vi "UHR-Fleezers Control (host) - 12.2.vi"() -> ()   [LabVIEW 2014] (continued)
      }
    }
    n3142 = Unbundle By Name(w3932) -> ("Y"=w3935:dbl[])
    n3143 = Unbundle By Name(w3929) -> ("Y"=w3938:dbl[])
    n3144 = Subtract(x=w3935, y=w3933) -> (x-y=w3936:dbl[])
    n3145 = Subtract(x=w3938, y=w3931) -> (x-y=w3937:dbl[])
    n3146 = Multiply(x=w3937, y="T2 a_x (nm/V)") -> (x*y=w3739:dbl[])
    n3147 = Multiply(x="T1 a_x (nm/V)", y=w3936) -> (x*y=w3740:dbl[])
    n3148 = Not(x="Trap Trig. Fl.") -> (.not. x?=w3776:bool)
    n3149 = Multiply(x=w3959, y=-1.0) -> (x*y=w3940:waveform(dbl))
    n3150 = Subtract(x=w3740, y=w3739) -> (x-y=w3928:dbl[])
    n3151 = Unbundle By Name(w3959) -> ("Y"=w3902:dbl[])
    n3152 = Unbundle By Name(w3960) -> ("Y"=w3741:dbl[])
    n3153 = Negate(x=w3928) -> (-x=w3737:dbl[])
    n3154 = Build Array(w3960, w3940) -> (→"Force":waveform(dbl)[])
    n3155 = Subtract(x=w3737, y="Offset (nm)") -> (x-y=w3900:dbl[])
    n3156 = case shown="True" "Read Lateness and Rel Phase" {
      tunnel: w3757 -> [w4306 w4330]
      tunnel: w3756 -> [w4307 w4329]
      tunnel: [w4306 w4328] -> w3926
      tunnel: [w4307 w4327] -> w3925
      frame False {
      }
      frame True {
        n3157 = xnode "Read/Write Control"("FPGA VI Reference In"=w4330, "error in"=w4329) -> ("FPGA VI Reference Out"=w4328:T22, "error out"=w4327:errorcluster, "GI Relative phase"=→"GI relative phase":i16, "Relative phase"=→"Relative phase (AI1)":i16, "AI Late Counter"=→"Late Counter (AI1)":u8, "GI Late Counter"=→"GI Late Counter":u8, "MCL Late Counter"=→"MCL Late Counter":u8, "MCL Relative Phase"=→"Relative Phase (MCL)":i16, "APD Acq Relative Phase"=→"APD Acq Relative Phase":i16, "APD 1 Gate Relative Phase"=→"APD 1 Gate Relative Phase":i16, "APD 2 Gate Relative Phase"=→"APD 2 Gate Relative Phase":i16, "APD Acq Late Counter"=→"APD Acq Late Counter":u8, "APD 1 Gate Late Counter"=→"APD 1 Gate Late Counter":u8, "APD 2 Gate Late Counter"=→"APD 2 Gate Late Counter":u8, "Green FB Relative Phase"=→"Relative phase (Green FB)":i16, "GI Relative phase 2"=→"GI relative phase 2":i16, "GI Late Counter 2"=→"GI Late Counter 2":u8, "Trap Pos FIFO Timeout"=→"Trap Pos FIFO Timeout":u16, "Trap AI FIFO Timeout"=→"Trap AI FIFO Timeout":u16, "RI relative phase"=→"RI relative phase":i16, "RI late counter"=→"RI late counter":u8)
      }
    }
    n3158 = call-poly <vilib>:"Mean.vi"("X"=w3902) -> ("mean"=w3743:dbl)  [unwired: 1 out]
    "T2 X" <- w3743
    n3159 = Negate(x=w3902) -> (-x=w3903:dbl[])
    n3160 = call-poly <vilib>:"Mean.vi"("X"=w3741) -> ("mean"=w3744:dbl)  [unwired: 1 out]
    "T1 X" <- w3744
    n3161 = Negate(x=w3743) -> (-x=w3742:dbl)
    n3162 = Bundle By Name(cluster=w3932, "Y"=w3900) -> (w3877:waveform(dbl))
    "Bead Separation" <- w3877
    n3163 = Add(x=w3741, y=w3903) -> (x+y=w3904:dbl[])
    n3164 = Add(x=w3744, y=w3742) -> (x+y=w3946:dbl)
    n3165 = Subtract(x=w3744, y=w3742) -> (x-y=→"Difference":dbl)
    n3166 = Divide(x=w3904, y=2.0) -> (x/y=→"Vec Mean of T1 T2":dbl[])
    n3167 = Divide(x=w3946, y=2.0) -> (x/y=w3906:dbl)
    "Mean" <- w3906
    n3168 = feedback-in #27("Trap Trig. Fl.") -> ()
    n3169 = feedback #27("Trap Trig. Fl.") -> (w3774:bool)
    n3170 = And(x=w3776, y=w3774) -> (x .and. y?=w3775:bool)
    n3171 = case "If have just turned off triggering" shown="True" w3775 {
      tunnel: w3757 -> [_ w4136]
      tunnel: w3756 -> [_ w4135]
      frame False {
      }
      frame True {
        w4134 = FALSE ("FPGA Trap Trig")
        n3172 = xnode "Read/Write Control"("FPGA VI Reference In"=w4136, "error in"=w4135, "FPGA Trap Trig"=w4134) -> ("FPGA VI Reference Out"=w4133:T22, "error out"=w4132:errorcluster)
        n3173 = xnode "Read/Write Control"("FPGA VI Reference In"=w4133, "error in"=w4132, "TTrig?"=w4134) -> ()  [unwired: 2 out]
        n3174 = local write "Initializing"(FALSE ("Initializing")) -> ()
        n3175 = local write "Triggered"(FALSE ("Triggered")) -> ()
        n3176 = local write "Waiting"(FALSE ("Waiting")) -> ()
      }
    }
    n3177 = Not(x=w3774) -> (.not. x?=w3787:bool)
    n3178 = And(x="Trap Trig. Fl.", y=w3787) -> (x .and. y?=w3784:bool)
    n3179 = local read "Tether"() -> (w3907:bool)
    n3180 = Or(x=w3784, y="Reinitialize") -> (x .or. y?=w3770:bool)
    n3181 = feedback #28(w3780) -> (w3785:string)
    n3182 = Select(t=w3780, s=w3784, f=w3785) -> (s? t:f=w3779:string)
    n3183 = Select(t=w3780, s="Reinitialize", f=w3779) -> (s? t:f=w3778:string)
    n3184 = feedback #29(0) -> (w3782:i32)
    n3185 = feedback #30(w3900) -> (w3899:dbl[])
    n3186 = Build Array (concatenate)(w3900, w3899) -> (w3738:dbl[])
    n3187 = case "For determining if there is a tether still" shown="True" w3907 {
      tunnel: w3906 -> [_ w4260]
      frame False {
      }
      frame True {
        n3188 = Greater?(x="Lost Tether Alarm Threshold (pN)", y=w4260) -> (0:w4258:bool)
        n3189 = case shown="True" w4258 {
          frame False {
          }
          frame True {
            w4261 = TRUE
            w4265 = FALSE ("Multiple tether")
            w4266 = FALSE ("Value (Signaling)")
            n3190 = flat-sequence {
              frame #0 {
                # "stop only if saving"
                n3191 = local read "Saving..."() -> (w4278:bool)
                n3192 = And(x=w4278, y="TA Cancel Save?") -> (x .and. y?=w4277:bool)
                n3193 = local write "Stop Saving"(w4277) -> ()
              }
              frame #1 {
                n3194 = case shown="True" "TA Green Off?" {
                  frame False {
                  }
                  frame True {
                    w4281 = FALSE ("Fl. Triggered...")
                    n3195 = local write "Fl. Triggered..."(w4281) -> ()
                    n3196 = property on="Green ON/Interlacing" class="Bool (strict)"("Val(Sgnl)"=w4281) -> ()  [unwired: 2 in, 2 out]
                  }
                }
              }
            }
            n3197 = local read "Time tether formed"() -> (w4272:timestamp)
            n3198 = Get Date/Time In Seconds() -> (seconds since 1Jan1904=w4273:timestamp)
            n3199 = Subtract(x=w4273, y=w4272) -> (x-y=w4271:dbl)
            n3200 = Number To Decimal String(number=w4271) -> (decimal integer string=w4268:string)  [unwired: 1 out]
            n3201 = local read "Messages"() -> (w4275:string)
            n3202 = call <vilib>:"Beep.vi"("use system alert? (T)"=FALSE, "duration (msec)"=u32 200, "frequency (Hz)"=u32 200) -> ()  [unwired: 9 out]
            n3203 = Concatenate Strings("Lost tether (" ("Message to add"), w4268, " s)." ("string")) -> (w4270:string)
            n3204 = local write "Tether"(FALSE ("Tether")) -> ()
            n3205 = call "Update messages.vi"("Message to add"=w4270, "Old message string"=w4275) -> ("New message string"=w4274:string)
            n3206 = local write "Messages"(w4274) -> ()
            n3207 = local write "Pause dwell"(w4266) -> ()
            n3208 = property on="Fl. Triggered..." class="Bool (strict)"("Val(Sgnl)"=w4266) -> ()  [unwired: 2 in, 2 out]
            n3209 = local write "Dip for Protein"(w4266) -> ()
            n3210 = property on="Trap Pos. FB ON" class="Bool (strict)"("Val(Sgnl)"=w4266) -> ()  [unwired: 2 in, 2 out]
            n3211 = property on="Trap Trig. Fl." class="Bool (strict)"("Val(Sgnl)"=w4266) -> ()  [unwired: 2 in, 2 out]
            n3212 = local write "Multiple tether"(w4265) -> ()
            n3213 = local write "Bad fit"(w4265) -> ()
            n3214 = local write "Hysteresis"(w4265) -> ()
            n3215 = local write "Good tether"(w4265) -> ()
            n3216 = local write "Save scans"(w4261) -> ()
            n3217 = local write "Restart DMA? (AOD)"(w4261) -> ()
          }
        }
      }
    }
    n3218 = case "For triggering actions based on the trap position (e.g., turning the excitation laser on if trap under feedback moves so far)" shown="True" "Trap Trig. Fl." {
      tunnel: w3765 -> [_ w4149]
      tunnel: w3778 -> [_ w4148]
      tunnel: ["" ("t") w4147] -> w3786
      tunnel: w3770 -> [_ w4146]
      tunnel: [0 ("t") w4145] -> w3783
      tunnel: w3782 -> [_ w4144]
      tunnel: w3757 -> [_ w4143]
      tunnel: w3756 -> [_ w4142]
      frame False {
      }
      frame True {
        n3219 = case shown="\"Wait for trigger\"" w4148 {
          tunnel: w4149 -> [w4166 _ _ w4214]
          tunnel: [w4163 w4195 "" ("t") w4217] -> w4147
          tunnel: w4146 -> [_ _ _ w4205]
          tunnel: [w4162 w4192 0 ("t") w4206] -> w4145
          tunnel: w4144 -> [_ w4194 _ w4212]
          tunnel: w4143 -> [w4151 w4189 _ w4208]
          tunnel: w4142 -> [w4150 w4188 _ w4207]
          frame "Wait for trigger" {
            n3220 = local read "Trap Trig. (FPGA)"() -> (w4154:bool)
            n3221 = Subtract(x=w4166, y="Mean T1 Position\nto compare (nm)") -> (x-y=w4159:dbl[])
            n3222 = call <vilib>:"Std Deviation and Variance.vi"("X"=w4159) -> ("mean"=→"mean":dbl, "standard deviation"=→"standard\ndeviation":dbl)  [unwired: 1 in, 1 out]
            n3223 = Array Max & Min(array=w4159) -> (max value=→"max value":dbl, min value=→"min value":dbl)  [unwired: 2 out]
            n3224 = Greater?(x=w4159, y="Threshold (nm)") -> (0:w4169:bool[])
            n3225 = case shown="True" w4154 {
              tunnel: w4151 -> [_ w4175]
              tunnel: w4150 -> [_ w4174]
              tunnel: [FALSE ("TTrig?") w4173] -> w4157
              frame False {
              }
              frame True {
                n3226 = xnode "Read/Write Control"("FPGA VI Reference In"=w4175, "error in"=w4174) -> ("TTrig?"=w4173:bool)  [unwired: 2 out]
              }
            }
            n3227 = Or Array Elements(Boolean array=w4169) -> (logical OR=w4156:bool)
            n3228 = Select(t=w4157, s=w4154, f=w4156) -> (s? t:f=w4155:bool)
            n3229 = Not(x=w4154) -> (.not. x?=w4153:bool)
            n3230 = And(x=w4155, y=w4153) -> (x .and. y?=w4152:bool)
            n3231 = Select(t="Triggered", s=w4155, f="Wait for trigger") -> (s? t:f=w4163:string)
            n3232 = case shown="True" w4155 {
              tunnel: [0 0] -> w4162
              tunnel: w4151 -> [_ w4180]
              tunnel: w4150 -> [_ w4179]
              frame False {
                "Waiting" <- TRUE ("Waiting")
              }
              frame True {
                n3233 = xnode "Read/Write Control"("FPGA VI Reference In"=w4180, "error in"=w4179, "TTrig?"=FALSE) -> ()  [unwired: 2 out]
                n3234 = local read "Messages"() -> (w4183:string)
                n3235 = call <vilib>:"Beep.vi"() -> ()  [unwired: 12 in]
                n3236 = call "Update messages.vi"("Message to add"="Unwinding trigger.", "Old message string"=w4183) -> ("New message string"=w4184:string)
                n3237 = local write "Messages"(w4184) -> ()
                n3238 = local write "Waiting"(FALSE ("Waiting")) -> ()
                "Triggered" <- TRUE ("Triggered")
              }
            }
            n3239 = case "Only need to turn on laser if host triggered" shown="True" w4152 {
              frame False {
              }
              frame True {
                n3240 = property on="Green ON/Interlacing" class="Bool (strict)"("Val(Sgnl)"=TRUE ("Value (Signaling)")) -> ()  [unwired: 2 in, 2 out]
              }
            }
          }
          frame "Triggered" {
            n3241 = local read "Trap Trig. (FPGA)"() -> (w4191:bool)
            n3242 = Increment(x=w4194) -> (x+1=w4192:i32)
            n3243 = Greater Or Equal?(x=w4192, y="Fl. ON time (n)") -> (x >= y?=w4190:bool)
            n3244 = Select(t="Wait for trigger", s=w4190, f="Triggered" ("t")) -> (s? t:f=w4195:string)
            n3245 = And(x=w4190, y=w4191) -> (x .and. y?=w4187:bool)
            n3246 = case shown="True" w4187 {
              tunnel: w4189 -> [_ w4199]
              tunnel: w4188 -> [_ w4198]
              frame False {
              }
              frame True {
                n3247 = xnode "Read/Write Control"("FPGA VI Reference In"=w4199, "error in"=w4198, "FPGA Trap Trig"=TRUE) -> ()  [unwired: 2 out]
              }
            }
            n3248 = case shown="True" w4190 {
              frame False {
              }
              frame True {
                w4201 = FALSE ("Value (Signaling)")
                n3249 = local write "Triggered"(w4201) -> ()
                n3250 = local write "Waiting"(TRUE ("Waiting")) -> ()
                n3251 = property on="Green ON/Interlacing" class="Bool (strict)"("Val(Sgnl)"=w4201) -> ()  [unwired: 2 in, 2 out]
              }
            }
          }
          frame "Do nothing" {
          }
          frame "Initialize", Default {
            n3252 = Increment(x=w4212) -> (x+1=w4216:i32)
            n3253 = Select(t=1, s=w4205, f=w4216) -> (s? t:f=w4206:i32)
            n3254 = feedback #31(w4214) -> (w4220:dbl[])
            n3255 = Build Array (concatenate)(w4214, w4220) -> (w4213:dbl[])
            n3256 = Greater Or Equal?(x=w4206, y="Wait to get offset (n)") -> (x >= y?=w4209:bool)
            n3257 = Select(t=w4214, s=w4205, f=w4213) -> (s? t:f=w4215:dbl[])
            n3258 = feedback-in #31(w4215) -> ()
            n3259 = call-poly <vilib>:"Mean.vi"("X"=w4215) -> ("mean"=w4210:dbl)  [unwired: 1 out]
            n3260 = local write "Mean T1 Position\nto compare (nm)"(w4210) -> ()
            n3261 = case shown="True" w4205 {
              tunnel: w4208 -> [_ w4226]
              tunnel: w4207 -> [_ w4225]
              frame False {
              }
              frame True {
                w4222 = FALSE ("FPGA Trap Trig")
                n3262 = xnode "Read/Write Control"("FPGA VI Reference In"=w4226, "error in"=w4225, "FPGA Trap Trig"=w4222) -> ("FPGA VI Reference Out"=w4224:T22, "error out"=w4223:errorcluster)
                n3263 = xnode "Read/Write Control"("FPGA VI Reference In"=w4224, "error in"=w4223, "TTrig?"=w4222) -> ()  [unwired: 2 out]
              }
            }
            n3264 = Select(t="Wait for trigger", s=w4209, f="Initialize") -> (s? t:f=w4217:string)
            n3265 = case shown="True" w4209 {
              tunnel: w4210 -> [_ w4229]
              tunnel: w4208 -> [_ w4238]
              tunnel: w4207 -> [_ w4237]
              frame False {
                n3266 = local write "Waiting"(FALSE ("Waiting")) -> ()
                "Initializing" <- TRUE ("Initializing")
              }
              frame True {
                n3267 = local read "Threshold (nm)"() -> (w4241:dbl)
                n3268 = local read "AOM X Cal (nm/MHz)"() -> (w4240:dbl)
                n3269 = Add(x=w4229, y=w4241) -> (x+y=w4242:dbl)
                n3270 = Divide(x=w4242, y=w4240) -> (x/y=w4239:dbl)
                n3271 = call "IR AOM freq to word.vi"("Frequency In (MHz)"=w4239) -> ("Frequency Word Out (double)"=w4236:dbl)
                n3272 = local write "Initializing"(FALSE ("Initializing")) -> ()
                n3273 = local write "Waiting"(TRUE ("Waiting")) -> ()
                n3274 = To Quad Integer(1:w4236) -> (0:w4235:i64)
                n3275 = xnode "Read/Write Control"("FPGA VI Reference In"=w4238, "error in"=w4237, "FPGA TTrig Thresh"=w4235) -> ("FPGA VI Reference Out"=w4232:T22, "error out"=w4231:errorcluster)
                n3276 = xnode "Read/Write Control"("FPGA VI Reference In"=w4232, "error in"=w4231, "FPGA Trap Trig"=TRUE) -> ()  [unwired: 2 out]
              }
            }
          }
        }
      }
    }
    n3277 = feedback-in #28(w3786) -> ()
    n3278 = feedback-in #29(w3783) -> ()
    n3279 = Split 1D Array(array=w3738, index=w3800) -> (first subarray=w3896:dbl[])  [unwired: 1 out]
    n3280 = feedback-in #30(w3896) -> ()
    n3281 = call-poly <vilib>:"Mean.vi"("X"=w3896) -> ("mean"=w3895:dbl)  [unwired: 1 out]
    "Bead Mean (nm)" <- w3895
    n3282 = Subtract(x=w3896, y=w3895) -> (x-y=w3894:dbl[])
    n3283 = Square(x=w3894) -> (x^2=w3893:dbl[])
    n3284 = call-poly <vilib>:"Mean.vi"("X"=w3893) -> ("mean"=w3892:dbl)  [unwired: 1 out]
    n3285 = Square Root(x=w3892) -> (sqrt(x)=w3891:dbl)
    n3286 = Multiply(x=10.0, y=w3891) -> (x*y=→"RMS (Å)":dbl)
    n3287 = xnode ("Read/Write Control")("FPGA VI Reference In"=w3926, "error in"=w3925) -> ("FPGA VI Reference Out"=w3768:T22, "error out"=w3767:errorcluster, "AI2 Y Sum Set 1"=w4021:i16, "AI2 Y Sum Set 2"=w4020:i16, "AI1 X Set 1"=w3828:fxp<+/-,16,1>, "AI1 X Set 2"=w3827:fxp<+/-,16,1>, "Trap Pos FB Int Signal"=→"Trap Pos FB Int Signal":fxp<+/-,24,9>, "Trap Pos FB Int-Norm Signal"=→"Trap Pos FB Int-Norm Signal":fxp<+/-,16,1>, "Trap Pos FB Action"=w3821:i64, "Scanning"=→"AOD Scanning":bool, "Scan I"=→"AOD Scan I":u64, "Scanning MCL"=w4023:bool, "Scan I (MCL)"=→"MCL Scan I":u64, "Green FB Sum"=w3963:i16, "Trap Pos FB Action"=w3755:i64, "Wiggling 1"=→"Wiggling T1":bool, "TTrig Fin Thresh"=w3751:i64, "Wiggling 2"=→"Wiggling T2":bool, "Red FB Sum"=w3718:i16)  [unwired: 2 out]
    "MCL Scanning" <- w4023
    "Trap Pos FB Action" <- w3821
    n3288 = local read "FB Trig Integrate"() -> (w3749:u32)
    n3289 = Divide(x=w3963, y=3276.7) -> (x/y=w3717:dbl)
    "Green laser intensity (V)" <- w3717
    n3290 = Divide(x=w3718, y=3276.7) -> (x/y=w3716:dbl)
    "Red laser intensity (V)" <- w3716
    n3291 = Divide(x=w3755, y=w3749) -> (x/y=w3748:dbl)
    "TTrig Sig (Int)" <- w3748
    n3292 = Divide(x=w3751, y=w3749) -> (x/y=w3746:dbl)
    "TTrig Fin Thresh (Int)" <- w3746
    n3293 = local read "AOM X Cal (nm/MHz)"() -> (w3754:dbl)
    n3294 = local read "AI2 (V)"() -> (w4022:cluster{"Set 1":dbl, "Set 2":dbl})
    n3295 = Bundle By Name(cluster=w4022, "Set 1"=w4021, "Set 2"=w4020) -> (w4018:cluster{"Set 1":dbl, "Set 2":dbl})
    n3296 = Divide(x=w3821, y=327.67) -> (x/y=w3733:dbl)
    n3297 = local read "Trap X (AI1)"() -> (w3841:T10)
    n3298 = Bundle(w3717, w3716) -> (→"Excitation laser intensities plot":cluster{dbl, dbl})  [unwired: 1 in]
    n3299 = call "IR AOM word double to freq.vi"("Frequency Word In (double)"=w3746) -> ("Frequency Out (MHz)"=w3745:dbl)
    n3300 = call "IR AOM word double to freq.vi"("Frequency Word In (double)"=w3748) -> ("Frequency Out (MHz)"=w3747:dbl)
    n3301 = Divide(x=w4018, y=3276.7) -> (x/y=w4017:cluster{"Set 1":dbl, "Set 2":dbl})
    n3302 = Multiply(x=w3747, y=w3754) -> (x*y=w3753:dbl)
    "TTrig Sig (nm)" <- w3753
    n3303 = Multiply(x=w3745, y=w3754) -> (x*y=w3752:dbl)
    "TTrig Fin Thresh (nm)" <- w3752
    n3304 = local write "AI2 (V)"(w4017) -> ()
    n3305 = local read "Trap Pos. FB Range"() -> (w3732:T12)
    n3306 = Bundle(cluster=w3841, "Trap 1"=w3828, "Trap 2"=w3827) -> (→"Trap X (AI1)":T10)
    n3307 = Bundle(w3753, w3752) -> (→"TTrig":cluster{dbl, dbl})  [unwired: 1 in]
    n3308 = Unbundle(w3732) -> ("output high"=w3731:fxp<+/-,64,32>)  [unwired: 1 out]
    n3309 = Divide(x=w3733, y=w3731) -> (x/y=→"Action (%)":dbl)
    n3310 = flat-sequence "To save data" {
      tunnel: [w5105] -> w4040
      tunnel: [w5106] -> w4039
      tunnel: w3993 -> [w5078]
      tunnel: w3773 -> [w5103]
      tunnel: ["Save Calibration"] -> w4014
      tunnel: w4011 -> [w5102]
      tunnel: [w5096] -> w4010
      tunnel: [w5093] -> w4009
      tunnel: [w5090] -> w4008
      tunnel: w3992 -> [w5092]
      tunnel: w3910 -> [w5086]
      tunnel: [w5086] -> w3909
      tunnel: ["Start Saving"] -> w3879
      tunnel: [w5080] -> w3813
      tunnel: [w5079] -> w3812
      tunnel: [w5075] -> w3697
      tunnel: w4040 -> [w5380]
      tunnel: w4039 -> [w5379]
      tunnel: w3814 -> [w5378]
      tunnel: w4014 -> [w5377]
      tunnel: w4010 -> [w5375]
      tunnel: w4009 -> [w5374]
      tunnel: w4008 -> [w5373]
      tunnel: w3888 -> [w5372]
      tunnel: w3919 -> [w5371]
      tunnel: w3909 -> [w5370]
      tunnel: w3879 -> [w5369]
      tunnel: w3877 -> [w5368]
      tunnel: w3855 -> [w5367]
      tunnel: w3813 -> [w5366]
      tunnel: w3812 -> [w5365]
      tunnel: w3811 -> [w5364]
      tunnel: w3734 -> [w5363]
      tunnel: w3697 -> [w5362]
      frame #0 {
        n3311 = Or(x="Save N Sets", y="Start Saving") -> (x .or. y?=w5087:bool)
        n3312 = To Double Precision Float(number=w5102) -> (double precision float=w5097:dbl)
        n3313 = Build Array(w5087, "Save Calibration", w5078, w5092) -> (w5101:bool[])
        n3314 = Compound Arithmetic op=OR("Save Calibration", w5078, w5087, w5092) -> (w5104:bool)
        n3315 = Boolean Array To Number(Boolean array=w5101) -> (number=w5099:u32)
        n3316 = feedback #32(FALSE ("Save APD Data\nwith Trap Data")) -> (w5081:bool)
        n3317 = feedback #33(refnum<k0> refnum) -> (w5076:refnum<file>)
        n3318 = feedback #34(refnum<k0> refnum) -> (w5107:refnum<file>)
        n3319 = feedback #35(refnum<k0> refnum) -> (w5083:refnum<file>)
        n3320 = feedback #36(FALSE ("Save APD Data\nwith Trap Data")) -> (w5091:bool)
        n3321 = feedback #37(refnum<k0> refnum) -> (w5094:refnum<file>)
        n3322 = feedback #38(0) -> (w5109:i32)
        n3323 = feedback #39() -> (w5098:u32)  [unwired: 1 out]
        n3324 = case shown="True" w5104 {
          tunnel: [w5117 1] -> w5105
          tunnel: w5109 -> [w5119 _]
          tunnel: [w5118 w5139] -> w5106
          tunnel: w5107 -> [w5118 _]
          tunnel: w5103 -> [_ w5159]
          tunnel: w5097 -> [_ w5157]
          tunnel: w5099 -> [_ w5160]
          tunnel: [w5116 w5138] -> w5096
          tunnel: w5098 -> [w5116 _]
          tunnel: [w5115 w5136] -> w5093
          tunnel: w5094 -> [w5115 _]
          tunnel: [w5114 w5135] -> w5090
          tunnel: w5091 -> [w5114 _]
          tunnel: "Start Saving" -> [_ w5133]
          tunnel: w5086 -> [_ w5132]
          tunnel: [w5113 w5124] -> w5079
          tunnel: w5083 -> [w5113 _]
          tunnel: [w5112 w5122] -> w5080
          tunnel: w5081 -> [w5112 _]
          tunnel: w5076 -> [w5111 _]
          tunnel: [w5111 w5121] -> w5075
          frame False {
            n3325 = Increment(x=w5119) -> (x+1=w5117:i32)
          }
          frame True {
            w5129 = FALSE ("Start Saving")
            w5134 = 9.0  # File Version
            w5142 = FALSE ("prepend array or string size? (T)")
            w5140 = T29."big-endian, network order" ("byte order (0:big-endian, network order)")
            n3326 = local read "BD 1 Frequency 1 (MHz)"() -> (w5156:dbl)
            n3327 = local read "BD 2 Frequency 1 (MHz)"() -> (w5155:dbl)
            n3328 = local read "BD 1 Frequency 2 (MHz)"() -> (w5154:dbl)
            n3329 = local read "BD 2 Frequency 2 (MHz)"() -> (w5153:dbl)
            n3330 = local read "BD 1 Frequency 3 (MHz)"() -> (w5152:dbl)
            n3331 = local read "BD 2 Frequency 3 (MHz)"() -> (w5151:dbl)
            n3332 = Array Size(array=w5132) -> (size(s)=w5131:i32)
            n3333 = To Double Precision Float(number=w5131) -> (double precision float=w5130:dbl)
            n3334 = Build Array("Save APD Data\nwith Trap Data", "Save Trap Pos. Data") -> (w5126:bool[])
            n3335 = Boolean Array To Number(Boolean array=w5126) -> (number=w5125:u32)
            n3336 = Build Array(w5156, w5155, w5154, w5153, w5152, w5151) -> (w5150:dbl[])
            n3337 = case shown="4" w5160 {
              tunnel: w5159 -> [w5261 w5284 w5301 w5340]
              tunnel: w5130 -> [w5266 w5291 w5321 w5359]
              tunnel: w5157 -> [w5265 w5290 w5320 w5358]
              tunnel: [w5262 w5286 w5312 w5350] -> w5148
              tunnel: [w5254 "Cal sets to save" w5302 w5341] -> w5138
              tunnel: w5150 -> [w5263 w5287 w5314 w5352]
              tunnel: "Save APD Data\nwith Trap Data" -> [w5260 _ w5298 w5338]
              tunnel: [w5260 FALSE ("Save APD Data\nwith Trap Data") w5298 w5338] -> w5135
              tunnel: w5134 -> [w5257 w5281 w5296 w5336]
              tunnel: w5133 -> [w5256 _ _ _]
              tunnel: [w5243 "Active cal?" w5295 w5326] -> w5122
              tunnel: "Save Trap Pos. Data" -> [w5243 _ w5295 w5326]
              tunnel: w5125 -> [w5248 _ w5294 w5325]
              tunnel: [w5243 w5275 w5293 w5324] -> w5120
              frame 1, Default {
                # "timeseries"
                n3338 = case shown="True" "Profile" {
                  tunnel: [w5269 w5273] -> w5252
                  tunnel: [w5269 w5272] -> w5251
                  tunnel: [w5269 w5271] -> w5250
                  tunnel: [w5269 w5270] -> w5249
                  frame False {
                    w5269 = 0.0 ("f")
                  }
                  frame True {
                    n3339 = local read "Current Position"() -> (w5274:cluster{dbl, dbl, dbl})
                    n3340 = local read "Y change (mm)"() -> (w5270:dbl)
                    n3341 = Unbundle(w5274) -> (w5273:dbl, w5272:dbl, w5271:dbl)
                  }
                }
                n3342 = local read "Save ave N"() -> (w5268:dbl)
                n3343 = Multiply(x=w5268, y=w5261) -> (x*y=w5267:dbl)
                n3344 = To Double Precision Float(number=w5248) -> (double precision float=w5259:dbl)
                n3345 = Select(t=4.0, s="Profile", f=0.0) -> (s? t:f=w5244:dbl)
                n3346 = Build Array(w5257, w5261, w5267, w5266, w5265, w5244) -> (w5264:dbl[])
                n3347 = Build Array(w5259, w5252, w5251, w5250, w5249) -> (w5258:dbl[])
                n3348 = Select(t=u32 4000000000, s=w5256, f="N sets to save") -> (s? t:f=w5254:u32)
                n3349 = Build Array (concatenate)(w5264, w5263, w5258) -> (w5262:dbl[])
              }
              frame 2 {
                w5275 = FALSE
                w5283 = 0.0 ("f")
                # "If doing active calibration,\nalso save trap position file"
                # "calibration"
                n3350 = property on="Wiggle" class="Bool (strict)"("Val(Sgnl)"="Active cal?") -> ()  [unwired: 2 in, 2 out]
                n3351 = Select(t=2.0, s="Active cal?", f=0.0) -> (s? t:f=w5277:dbl)
                n3352 = Build Array(w5277, w5283, w5283, w5283, w5283) -> (w5282:dbl[])
                n3353 = Build Array(w5281, w5284, w5284, w5291, w5290, 1.0 ("t")) -> (w5288:dbl[])
                n3354 = local write "Saving Move"(w5275) -> ()
                n3355 = Build Array (concatenate)(w5288, w5287, w5282) -> (w5286:dbl[])
                "Calibrating..." <- TRUE ("Calibrating...")
              }
              frame 4 {
                w5293 = FALSE
                w5299 = 0.0 ("f")
                # "scan dir (x/y = 0/1)"
                # "cycles/step"
                # "n scans (f/b)"
                # "steps"
                # "freq. range"
                # "AOD raster scan"
                n3356 = local read "Number of F/B Scans (AOD)"() -> (w5306:u16)
                n3357 = local read "Cycles/step (AOD)"() -> (w5308:u64)
                n3358 = local read "Scan Range (MHz)"() -> (w5311:dbl)
                n3359 = local read "Scan steps (AOD)"() -> (w5310:u64)
                n3360 = local read "Scan BD"() -> (w5318:bool)
                n3361 = local read "Save ave N"() -> (w5323:dbl)
                n3362 = Boolean To (0,1)(Boolean=w5318) -> (0, 1=w5317:i16)
                n3363 = To Double Precision Float(number=w5306) -> (double precision float=w5305:dbl)
                n3364 = To Double Precision Float(number=w5310) -> (double precision float=w5309:dbl)
                n3365 = To Double Precision Float(number=w5308) -> (double precision float=w5307:dbl)
                n3366 = To Double Precision Float(number=w5317) -> (double precision float=w5316:dbl)
                n3367 = Multiply(x=w5323, y=w5301) -> (x*y=w5322:dbl)
                n3368 = To Double Precision Float(number=w5294) -> (double precision float=w5300:dbl)
                n3369 = Build Array(w5300, w5299, w5299, w5299, w5299) -> (w5297:dbl[])
                n3370 = local read "N sets should be saved"() -> (w5303:dbl)
                n3371 = local write "Raster Scanning..."(w5293) -> ()
                n3372 = Build Array(w5316, w5311, w5309, w5307, w5305) -> (w5313:dbl[])
                n3373 = Build Array(w5296, w5301, w5322, w5321, w5320, 2.0 ("t")) -> (w5315:dbl[])
                n3374 = local write "Saving Move"(w5293) -> ()
                n3375 = Round Toward +Infinity(x=w5303) -> (ceil(x): smallest int >= x=w5304:dbl)
                n3376 = Build Array (concatenate)(w5315, w5314, w5297, w5313) -> (w5312:dbl[])
                n3377 = To Unsigned Long Integer(number=w5304) -> (unsigned 32bit integer=w5302:u32)
              }
              frame 8 {
                w5324 = FALSE
                w5333 = 0.0 ("f")
                # "MCL raster scan"
                n3378 = local read "Number of scans (MCL)"() -> (w5328:u64)
                n3379 = local write "Saving Move"(w5324) -> ()
                n3380 = local read "Scan lines (y)"() -> (w5327:u64)
                n3381 = local read "2D or 1D Scan"() -> (w5330:bool)
                n3382 = local read "Scan Range (V)\n(of steps)"() -> (w5349:dbl)
                n3383 = local read "Fast Scan Dir"() -> (w5356:bool)
                n3384 = local read "Cycles/step (MCL)"() -> (w5346:u64)
                n3385 = local read "Scan steps (MCL)"() -> (w5348:u64)
                n3386 = Select(t=w5327, s=w5330, f=w5328) -> (s? t:f=w5329:u64)
                n3387 = Boolean To (0,1)(Boolean=w5330) -> (0, 1=w5332:i16)
                n3388 = local read "Save ave N"() -> (w5361:dbl)
                n3389 = local read "Initial X"() -> (w5335:dbl)
                n3390 = local read "Initial Y"() -> (w5334:dbl)
                n3391 = To Double Precision Float(number=w5332) -> (double precision float=w5331:dbl)
                n3392 = Boolean To (0,1)(Boolean=w5356) -> (0, 1=w5355:i16)
                n3393 = To Double Precision Float(number=w5329) -> (double precision float=w5344:dbl)
                n3394 = To Double Precision Float(number=w5348) -> (double precision float=w5347:dbl)
                n3395 = To Double Precision Float(number=w5346) -> (double precision float=w5345:dbl)
                n3396 = To Double Precision Float(number=w5355) -> (double precision float=w5354:dbl)
                n3397 = Multiply(x=w5361, y=w5340) -> (x*y=w5360:dbl)
                n3398 = To Double Precision Float(number=w5325) -> (double precision float=w5339:dbl)
                n3399 = local read "N sets should be saved (MCL)"() -> (w5342:dbl)
                n3400 = Build Array(w5339, w5331, w5333, w5333, w5333) -> (w5337:dbl[])
                n3401 = Build Array(w5354, w5349, w5347, w5345, w5344, w5335, w5334) -> (w5351:dbl[])
                n3402 = Build Array(w5336, w5340, w5360, w5359, w5358, 3.0 ("t")) -> (w5353:dbl[])
                n3403 = Round Toward +Infinity(x=w5342) -> (ceil(x): smallest int >= x=w5343:dbl)
                n3404 = Build Array (concatenate)(w5353, w5352, w5337, w5351) -> (w5350:dbl[])
                n3405 = To Unsigned Long Integer(number=w5343) -> (unsigned 32bit integer=w5341:u32)
              }
            }
            n3406 = local read "Index"() -> (w5165:dbl)
            n3407 = call "Create new save file.vi"("Insert"="", "Ext"=".dat", "Index In"=w5165) -> ("Path Out"=w5123:path, "Index Out"=w5137:dbl)
            n3408 = case shown="True" w5120 {
              tunnel: w5123 -> [_ w5172]
              tunnel: [refnum<k0> refnum w5170] -> w5121
              frame False {
              }
              frame True {
                n3409 = Path To String(path=w5172) -> (string=w5181:string)
                n3410 = Get Date/Time In Seconds() -> (seconds since 1Jan1904=w5191:timestamp)
                n3411 = String Length(string=w5181) -> (length=w5186:i32)
                n3412 = Subtract(x=w5186, y=4) -> (x-y=w5185:i32)
                n3413 = String Subset(string=w5181, length (rest)=w5185) -> (substring=w5183:string)  [unwired: 1 in]
                n3414 = call <vilib>:"Space Constant.vi"() -> ("String"=w5187:string)
                n3415 = Format Date/Time String(time format string (%c)="%H:%M:%S%3u", seconds (now)=w5191, UTC format=TRUE) -> (date/time string=w5188:string)
                n3416 = Concatenate Strings(w5183, "_stagetime.txt") -> (w5182:string)
                n3417 = String To Path(string=w5182) -> (path=w5179:path)
                n3418 = Open/Create/Replace File(file path (use dialog)=w5179, operation (0:open)=T30."create", access (0:read/write)=enum16{"read/write", "read-only", "write-only"}."write-only") -> (refnum out=w5178:refnum<file>, error out=w5175:errorcluster)  [unwired: 3 in, 1 out]
                n3419 = Deny Access(4:w5175, 7:w5178) -> (3:w5177:refnum<file>)  [unwired: 1 in, 1 out]
                n3420 = local read "Raster Scanning..."() -> (w5194:bool)
                n3421 = Concatenate Strings(w5188, w5187, "start", "\r\n") -> (w5176:string)
                n3422 = local read "Calibrating..."() -> (w5193:bool)
                n3423 = local write "Move Time"(w5188) -> ()
                n3424 = Write to Text File(file (use dialog)=w5177, text=w5176) -> (refnum out=w5170:refnum<file>)  [unwired: 2 in, 2 out]
                n3425 = Or(x=w5194, y=w5193) -> (x .or. y?=w5196:bool)
                n3426 = Not(x=w5196) -> (.not. x?=w5195:bool)
                n3427 = local write "Saving Move"(w5195) -> ()
              }
            }
            n3428 = local write "Save Calibration"(w5129) -> ()
            n3429 = local write "Start Saving"(w5129) -> ()
            n3430 = local write "Save file name"(w5123) -> ()
            n3431 = local write "Index"(w5137) -> ()
            n3432 = local write "Save index"(w5137) -> ()
            n3433 = Array Size(array=w5148) -> (size(s)=w5149:i32)
            n3434 = Open/Create/Replace File(file path (use dialog)=w5123, operation (0:open)=T30."create", access (0:read/write)=enum16{"read/write", "read-only", "write-only"}."write-only") -> (refnum out=w5162:refnum<file>)  [unwired: 1 in, 4 out]
            n3435 = local write "Saving..."(TRUE ("Saving...")) -> ()
            n3436 = To Double Precision Float(number=w5149) -> (double precision float=w5147:dbl)
            n3437 = String Length(string="Comment (data description)") -> (length=w5145:i32)
            n3438 = To Double Precision Float(number=w5145) -> (double precision float=w5144:dbl)
            n3439 = Deny Access(7:w5162) -> (3:w5161:refnum<file>)  [unwired: 1 in, 2 out]
            n3440 = Build Array (concatenate)(w5147, w5148, w5144) -> (w5146:dbl[])
            n3441 = case "If fluorescence data to be saved" shown="True" w5135 {
              tunnel: w5123 -> [_ w5242]
              tunnel: [refnum<k0> refnum w5222] -> w5136
              frame False {
              }
              frame True {
                w5221 = 0.0
                n3442 = local read "APD Integration Time (s)"() -> (w5227:dbl)
                n3443 = local read "N APD Samp/step"() -> (w5220:dbl)
                n3444 = Path To String(path=w5242) -> (string=w5241:string)
                n3445 = String Length(string=w5241) -> (length=w5240:i32)
                n3446 = Subtract(x=w5240, y=4) -> (x-y=w5238:i32)
                n3447 = String Subset(string=w5241, length (rest)=w5238) -> (substring=w5237:string)  [unwired: 1 out]
                n3448 = Build Array(w5227, w5220, w5221, w5221, w5221, w5221, w5221, w5221) -> (w5224:dbl[])
                n3449 = Concatenate Strings(w5237, "_fl.dat" ("string")) -> (w5235:string)
                n3450 = Array Size(array=w5224) -> (size(s)=w5226:i32)
                n3451 = String To Path(string=w5235) -> (path=w5231:path)
                n3452 = Open/Create/Replace File(file path (use dialog)=w5231, operation (0:open)=T30."create", access (0:read/write)=enum16{"read/write", "read-only", "write-only"}."write-only") -> (refnum out=w5232:refnum<file>)  [unwired: 1 in, 4 out]
                n3453 = Deny Access(7:w5232) -> (3:w5228:refnum<file>)  [unwired: 1 in, 2 out]
                n3454 = To Double Precision Float(number=w5226) -> (double precision float=w5225:dbl)
                n3455 = Build Array (concatenate)(w5225, w5224) -> (w5223:dbl[])
                n3456 = Write to Binary File(file (use dialog)=w5228, data=w5223, 5:FALSE ("prepend array or string size? (T)"), 9:T29."big-endian, network order" ("byte order (0:big-endian, network order)")) -> (refnum out=w5222:refnum<file>)  [unwired: 1 in, 3 out]
              }
            }
            n3457 = case shown="True" w5122 {
              tunnel: w5123 -> [_ w5204]
              tunnel: [refnum<k0> refnum w5203] -> w5124
              frame False {
              }
              frame True {
                w5199 = 0.0 ("element")
                n3458 = Path To String(path=w5204) -> (string=w5218:string)
                n3459 = Build Array(w5199, w5199, w5199, w5199, w5199, w5199, w5199, w5199) -> (w5200:dbl[])
                n3460 = String Length(string=w5218) -> (length=w5217:i32)
                n3461 = Subtract(x=w5217, y=4) -> (x-y=w5215:i32)
                n3462 = Array Size(array=w5200) -> (size(s)=w5202:i32)
                n3463 = String Subset(string=w5218, length (rest)=w5215) -> (substring=w5214:string)  [unwired: 1 out]
                n3464 = To Double Precision Float(number=w5202) -> (double precision float=w5201:dbl)
                n3465 = Concatenate Strings(w5214, "_pos.dat" ("string")) -> (w5212:string)
                n3466 = Build Array (concatenate)(w5201, w5200) -> (w5198:dbl[])
                n3467 = String To Path(string=w5212) -> (path=w5208:path)
                n3468 = Open/Create/Replace File(file path (use dialog)=w5208, operation (0:open)=T30."create", access (0:read/write)=enum16{"read/write", "read-only", "write-only"}."write-only") -> (refnum out=w5209:refnum<file>)  [unwired: 1 in, 4 out]
                n3469 = Deny Access(7:w5209) -> (3:w5205:refnum<file>)  [unwired: 1 in, 2 out]
                n3470 = Write to Binary File(file (use dialog)=w5205, data=w5198, 5:FALSE ("prepend array or string size? (T)"), 9:T29."big-endian, network order" ("byte order (0:big-endian, network order)")) -> (refnum out=w5203:refnum<file>)  [unwired: 1 in, 3 out]
              }
            }
            n3471 = Write to Binary File(file (use dialog)=w5161, data=w5146, 5:w5142, 9:w5140) -> (refnum out=w5143:refnum<file>)  [unwired: 1 in, 3 out]
            n3472 = Write to Binary File(file (use dialog)=w5143, data="Comment (data description)", 5:w5142, 9:w5140) -> (refnum out=w5139:refnum<file>)  [unwired: 1 in, 3 out]
          }
        }
        n3473 = feedback-in #32(w5080) -> ()
        n3474 = feedback-in #33(w5075) -> ()
        n3475 = feedback-in #34(w5106) -> ()
        n3476 = feedback-in #35(w5079) -> ()
        n3477 = feedback-in #36(w5090) -> ()
        n3478 = feedback-in #37(w5093) -> ()
        n3479 = feedback-in #38(w5105) -> ()
        n3480 = feedback-in #39(w5096) -> ()
      }
      frame #1 {
        n3481 = local read "Saving..."() -> (w5376:bool)
        n3482 = case shown="True" w5376 {
          tunnel: w5380 -> [_ w5393]
          tunnel: w5379 -> [_ w5406]
          tunnel: w5378 -> [_ w5402]
          tunnel: w5377 -> [_ w5401]
          tunnel: w5375 -> [_ w5382]
          tunnel: w5374 -> [_ w5396]
          tunnel: w5373 -> [_ w5395]
          tunnel: w5372 -> [_ w5394]
          tunnel: w5371 -> [_ w5392]
          tunnel: w5370 -> [_ w5390]
          tunnel: w5369 -> [_ w5389]
          tunnel: w5368 -> [_ w5388]
          tunnel: w5367 -> [_ w5387]
          tunnel: w5366 -> [_ w5386]
          tunnel: w5365 -> [_ w5385]
          tunnel: w5364 -> [_ w5384]
          tunnel: w5363 -> [_ w5383]
          tunnel: w5362 -> [_ w5381]
          frame False {
          }
          frame True {
            n3483 = Multiply(x=w5393, y=w5392) -> (x*y=→"Time (s)":dbl)
            n3484 = Less Or Equal?(x=w5393, y=w5382) -> (x <= y?=w5404:bool)
            n3485 = Or(x="Stop Saving", y="Abort save 2") -> (x .or. y?=w5397:bool)
            n3486 = Not(x=w5397) -> (.not. x?=w5405:bool)
            n3487 = And(x=w5404, y=w5405) -> (x .and. y?=w5403:bool)
            n3488 = case shown="False" w5403 {
              tunnel: w5406 -> [w5416 w5503]
              tunnel: [0.0 w5506] -> w5400
              tunnel: w5393 -> [_ w5504]
              tunnel: w5382 -> [_ w5505]
              tunnel: w5402 -> [_ w5500]
              tunnel: w5401 -> [_ _]
              tunnel: w5396 -> [w5414 w5493]
              tunnel: w5395 -> [w5413 w5494]
              tunnel: w5394 -> [_ w5492]
              tunnel: w5390 -> [_ w5491]
              tunnel: w5389 -> [_ w5435]
              tunnel: w5388 -> [_ w5484]
              tunnel: w5387 -> [_ w5462]
              tunnel: w5386 -> [w5411 w5444]
              tunnel: w5385 -> [w5412 w5443]
              tunnel: w5384 -> [_ w5440]
              tunnel: w5383 -> [_ w5438]
              tunnel: w5381 -> [w5409 w5430]
              frame False {
                w5407 = FALSE
                n3489 = Close File(refnum=w5416) -> ()  [unwired: 1 in, 2 out]
                n3490 = case shown="True" w5413 {
                  tunnel: w5414 -> [_ w5428]
                  frame False {
                  }
                  frame True {
                    n3491 = Close File(refnum=w5428) -> ()  [unwired: 1 in, 2 out]
                  }
                }
                n3492 = case shown="True" w5411 {
                  tunnel: w5412 -> [_ w5427]
                  frame False {
                  }
                  frame True {
                    n3493 = Close File(refnum=w5427) -> ()  [unwired: 1 in, 2 out]
                  }
                }
                n3494 = local read "Saving Move"() -> (w5408:bool)
                n3495 = case shown="True" w5408 {
                  tunnel: w5409 -> [_ w5419]
                  frame False {
                  }
                  frame True {
                    n3496 = Get Date/Time In Seconds() -> (seconds since 1Jan1904=w5424:timestamp)
                    n3497 = call <vilib>:"Space Constant.vi"() -> ("String"=w5422:string)
                    n3498 = Format Date/Time String(time format string (%c)="%H:%M:%S%3u", seconds (now)=w5424, UTC format=TRUE) -> (date/time string=w5418:string)
                    n3499 = Concatenate Strings(w5418, w5422, "end") -> (w5420:string)
                    n3500 = Write to Text File(file (use dialog)=w5419, text=w5420) -> (refnum out=w5426:refnum<file>)  [unwired: 2 in, 2 out]
                    n3501 = Close File(refnum=w5426) -> ()  [unwired: 1 in, 2 out]
                    n3502 = property on="Move Time" class="Str"("Value"=w5418) -> ()  [unwired: 2 in, 2 out]
                    n3503 = local write "Saving Move"(FALSE) -> ()
                  }
                }
                n3504 = call <vilib>:"Beep.vi"() -> ()  [unwired: 3 in, 9 out]
                n3505 = local write "Raster Scanning..."(w5407) -> ()
                n3506 = local write "Calibrating..."(w5407) -> ()
                n3507 = property on="Abort wiggle" class="Bool (strict)"("Val(Sgnl)"=TRUE) -> ()  [unwired: 2 in, 2 out]
                n3508 = local write "Stop Saving"(w5407) -> ()
                "Saving..." <- w5407
              }
              frame True {
                n3509 = local read "Calibrating..."() -> (w5495:bool)
                n3510 = case "Write fl. data" shown="True" w5494 {
                  tunnel: w5493 -> [_ w5535]
                  tunnel: w5492 -> [_ w5534]
                  frame False {
                  }
                  frame True {
                    n3511 = Write to Binary File(file (use dialog)=w5535, data=w5534, 5:FALSE ("prepend array or string size? (T)"), 9:T29."big-endian, network order" ("byte order (0:big-endian, network order)")) -> ()  [unwired: 1 in, 4 out]
                  }
                }
                n3512 = Greater?(x="Save ave N", y=1.0) -> (0:w5498:bool)
                n3513 = Not(x=w5495) -> (.not. x?=w5497:bool)
                n3514 = local read "Saving Move"() -> (w5429:bool)
                n3515 = And(x=w5497, y=w5498) -> (x .and. y?=w5441:bool)
                n3516 = case shown="True" w5441 {
                  tunnel: w5440 -> [w5515 w5526]
                  tunnel: [w5515 w5518] -> w5439
                  tunnel: "Save ave N" -> [_ w5519]
                  frame False {
                  }
                  frame True {
                    w5516 = 2 ("dimension size")
                    n3517 = Array Size(array=w5526) -> (size(s)=w5520:i32)
                    n3518 = Divide(x=w5520, y=w5516) -> (x/y=w5524:dbl)
                    n3519 = Reshape Array(w5526, w5524, w5516) -> (w5525:u64[][])
                    n3520 = Transpose 2D Array(2D array=w5525) -> (transposed array=w5523:u64[][])
                    n3521 = for {
                      tunnel: w5523 -> [w5528] mode=indexing
                      tunnel: [w5527] -> w5517 mode=indexing
                      tunnel: w5519 -> [w5529]
                      workers-P: _ -> [_]
                      n3522 = call "downsample 1D array - U64.vi"("Ave N"=w5529, "Array In"=w5528) -> ("Array Out"=w5527:u64[])  [unwired: 1 in]
                    }
                    n3523 = Transpose 2D Array(2D array=w5517) -> (transposed array=w5522:u64[][])
                    n3524 = Divide(x=w5520, y=w5519) -> (x/y=w5521:dbl)
                    n3525 = Reshape Array(w5522, w5521) -> (w5518:u64[])
                  }
                }
                n3526 = case shown="True" w5441 {
                  tunnel: w5500 -> [w5538 w5550]
                  tunnel: [w5538 w5542] -> w5496
                  tunnel: "Save ave N" -> [_ w5543]
                  tunnel: w5491 -> [_ w5541]
                  frame False {
                  }
                  frame True {
                    n3527 = Array Size(array=w5550) -> (size(s)=w5544:i32)
                    n3528 = Array Size(array=w5541) -> (size(s)=w5540:i32)
                    n3529 = Divide(x=w5544, y=w5540) -> (x/y=w5548:dbl)
                    n3530 = Reshape Array(w5550, w5548, w5540) -> (w5549:i16[][])
                    n3531 = Transpose 2D Array(2D array=w5549) -> (transposed array=w5547:i16[][])
                    n3532 = for {
                      tunnel: w5547 -> [w5553] mode=indexing
                      tunnel: [w5552] -> w5539 mode=indexing
                      tunnel: w5543 -> [w5551]
                      workers-P: _ -> [_]
                      n3533 = call "downsample 1D array - I16.vi"("Ave N"=w5551, "Array In"=w5553) -> ("Array Out"=w5552:i16[])  [unwired: 1 out]
                    }
                    n3534 = Transpose 2D Array(2D array=w5539) -> (transposed array=w5546:i16[][])
                    n3535 = Divide(x=w5544, y=w5543) -> (x/y=w5545:dbl)
                    n3536 = Reshape Array(w5546, w5545) -> (w5542:i16[])
                  }
                }
                n3537 = case shown="True" w5429 {
                  tunnel: w5430 -> [_ w5510]
                  frame False {
                  }
                  frame True {
                    n3538 = event shown="[1] \"Move Time\": Value Change" {
                      selector: _ -> [_ _]
                      dyn-events: _ -> [_ _]
                      timeout: 1 -> [_ _]
                      tunnel: w5510 -> [_ w5511]
                      event Timeout {
                        n3539 = event-data() -> ()  [unwired: 1 in, 3 out]
                      }
                      event "Move Time": Value Change {
                        n3540 = event-data() -> ("NewVal"=w5514:string)  [unwired: 1 in, 5 out]
                        n3541 = Concatenate Strings(w5514, "\r\n") -> (w5512:string)
                        n3542 = Write to Text File(file (use dialog)=w5511, text=w5512) -> ()  [unwired: 2 in, 3 out]
                      }
                    }
                  }
                }
                n3543 = Index Array(array=w5462, index=1) -> (element=w5465:waveform(dbl))
                n3544 = Index Array(array=w5462, index=0) -> (element=w5467:waveform(dbl))
                n3545 = Unbundle By Name(w5465) -> ("Y"=w5469:dbl[])
                n3546 = Unbundle By Name(w5467) -> ("Y"=w5477:dbl[])
                n3547 = case "Write trap pos. data" shown="True" w5444 {
                  tunnel: w5443 -> [_ w5531]
                  tunnel: w5439 -> [_ w5530]
                  frame False {
                  }
                  frame True {
                    n3548 = Write to Binary File(file (use dialog)=w5531, data=w5530, 5:FALSE ("prepend array or string size? (T)"), 9:T29."big-endian, network order" ("byte order (0:big-endian, network order)")) -> ()  [unwired: 1 in, 4 out]
                  }
                }
                n3549 = Write to Binary File(file (use dialog)=w5503, data=w5496, 5:FALSE ("prepend array or string size? (T)"), 9:T29."big-endian, network order" ("byte order (0:big-endian, network order)")) -> ()  [unwired: 1 in, 4 out]
                n3550 = feedback #40(w5469) -> (w5471:dbl[])
                n3551 = Build Array (concatenate)(w5471, w5469) -> (w5470:dbl[])
                n3552 = Select(t=w5469, s=w5435, f=w5470) -> (s? t:f=w5455:dbl[])
                n3553 = feedback-in #40(w5455) -> ()
                n3554 = feedback #41(w5477) -> (w5490:dbl[])
                n3555 = Build Array (concatenate)(w5490, w5477) -> (w5489:dbl[])
                n3556 = Select(t=w5477, s=w5435, f=w5489) -> (s? t:f=w5464:dbl[])
                n3557 = feedback-in #41(w5464) -> ()
                n3558 = Divide(x=w5504, y=w5505) -> (x/y=w5507:dbl)
                n3559 = Multiply(x=w5507, y=100.0) -> (x*y=w5506:dbl)
                n3560 = Build Array(w5464, w5455) -> (→"Saved APD":dbl[][])
                n3561 = Array Size(array=w5464) -> (size(s)=w5482:i32)
                n3562 = Unbundle By Name(w5484) -> ("Y"=w5488:dbl[])
                n3563 = Subtract(x=w5482, y="N pts to average") -> (x-y=w5458:i32)
                n3564 = Multiply(x="N pts to average", y=u16 2) -> (x*y=w5459:u16)
                n3565 = Subtract(x=w5482, y=w5459) -> (x-y=w5457:i32)
                n3566 = feedback #42(w5488) -> (w5487:dbl[])
                n3567 = Build Array (concatenate)(w5487, w5488) -> (w5486:dbl[])
                n3568 = Select(t=w5488, s=w5435, f=w5486) -> (s? t:f=w5485:dbl[])
                "Trap Delta Graph" <- w5485
                n3569 = feedback-in #42(w5485) -> ()
                n3570 = Array Subset(array=w5464, index=w5458, length="N pts to average") -> (w5481:dbl[])
                n3571 = Array Subset(array=w5464, index=w5457, length="N pts to average") -> (w5480:dbl[])
                n3572 = Array Subset(array=w5455, index=w5458, length="N pts to average") -> (w5461:dbl[])
                n3573 = Array Subset(array=w5455, index=w5457, length="N pts to average") -> (w5460:dbl[])
                n3574 = Index Array(array=w5438, index=0) -> (element=w5436:waveform(dbl))
                n3575 = call-poly <vilib>:"Mean.vi"("X"=w5481) -> ("mean"=w5479:dbl)  [unwired: 1 out]
                n3576 = call-poly <vilib>:"Mean.vi"("X"=w5461) -> ("mean"=w5454:dbl)  [unwired: 1 out]
                n3577 = call-poly <vilib>:"Mean.vi"("X"=w5480) -> ("mean"=w5478:dbl)  [unwired: 1 out]
                n3578 = call-poly <vilib>:"Mean.vi"("X"=w5460) -> ("mean"=w5453:dbl)  [unwired: 1 out]
                n3579 = Unbundle By Name(w5436) -> ("Y"=w5433:dbl[])
                n3580 = Subtract(x=w5454, y=w5453) -> (x-y=w5445:dbl)
                "Delta Fl. 2" <- w5445
                n3581 = Subtract(x=w5479, y=w5478) -> (x-y=w5476:dbl)
                "Delta Fl. 1" <- w5476
                n3582 = Initialize Array(w5476, 1 ("dimension size")) -> (w5473:dbl[])
                n3583 = Initialize Array(w5445, 1 ("dimension size")) -> (w5450:dbl[])
                n3584 = feedback #43(w5473) -> (w5474:dbl[])
                n3585 = Build Array (concatenate)(w5474, w5473) -> (w5472:dbl[])
                n3586 = feedback #44(w5450) -> (w5451:dbl[])
                n3587 = Build Array (concatenate)(w5451, w5450) -> (w5449:dbl[])
                n3588 = feedback #45(w5433) -> (w5432:dbl[])
                n3589 = Build Array (concatenate)(w5432, w5433) -> (w5434:dbl[])
                n3590 = Select(t=w5433, s=w5435, f=w5434) -> (s? t:f=w5431:dbl[])
                "Saved trap pos" <- w5431
                n3591 = feedback-in #45(w5431) -> ()
                n3592 = Select(t=w5473, s=w5435, f=w5472) -> (s? t:f=w5448:dbl[])
                n3593 = feedback-in #43(w5448) -> ()
                n3594 = Select(t=w5450, s=w5435, f=w5449) -> (s? t:f=w5447:dbl[])
                n3595 = feedback-in #44(w5447) -> ()
                n3596 = Build Array(w5448, w5447) -> (→"Save APD Deriv":dbl[][])
              }
            }
            "Progress" <- w5400
            "Progress 2" <- w5400
          }
        }
      }
    }
    n3597 = local read "wait to reset values"() -> (w4025:bool)
    n3598 = Not(x=w4023) -> (.not. x?=w4026:bool)
    n3599 = And(x=w4026, y=w4025) -> (x .and. y?=w4027:bool)
    n3600 = case "Part of MCL raster scanning: returns to initial positions after scan done" shown="True" w4027 {
      tunnel: w3768 -> [w4896 w4903]
      tunnel: [w4896 w4902] -> w4029
      tunnel: w3767 -> [w4895 w4901]
      tunnel: [w4895 w4900] -> w4024
      frame False {
      }
      frame True {
        w4911 = 10.0 ("y")
        w4910 = 32767.0 ("y")
        # "to return scan values\nafter a synchronous \nAOM scan"
        n3601 = local read "AO2"() -> (w4904:dbl)
        n3602 = local read "AO1"() -> (w4905:dbl)
        n3603 = local write "wait to reset values"(FALSE ("wait to reset values")) -> ()
        n3604 = Multiply(x=w4905, y=w4910) -> (x*y=w4907:dbl)
        n3605 = Multiply(x=w4904, y=w4910) -> (x*y=w4909:dbl)
        n3606 = Divide(x=w4907, y=w4911) -> (x/y=w4906:dbl)
        n3607 = Divide(x=w4909, y=w4911) -> (x/y=w4908:dbl)
        n3608 = To Word Integer(number=w4906) -> (16bit integer=w4912:i16)
        n3609 = To Word Integer(number=w4908) -> (16bit integer=w4913:i16)
        n3610 = local read "Total Counts (ticks)"() -> (w4897:u32)
        n3611 = xnode "Read/Write Control"("FPGA VI Reference In"=w4903, "error in"=w4901, "AO1"=w4912, "AO2"=w4913, "MCL count"=w4897) -> ("FPGA VI Reference Out"=w4902:T22, "error out"=w4900:errorcluster)
        n3612 = local read "Scan Range (V)\n(of steps)"() -> (w4898:dbl)
        n3613 = property on="Scan Range (V)\n(of steps)" class="DigNum (strict)"("Val(Sgnl)"=w4898) -> ()  [unwired: 2 in, 2 out]
      }
    }
    n3614 = node-c288() -> ()  [unwired: 2 out]
  }
  n3615 = VISA Close(VISA resource name=w129, error in (no error)=w128) -> (error out=w172:errorcluster)
  n3616 = call <vilib>:"Simple Error Handler.vi"("error in (no error)"=w172) -> ()  [unwired: 1 in, 8 out]
  n3617 = node-c288(w134) -> ()  [unwired: 1 out]
  n3618 = node-c288(w216) -> ()  [unwired: 1 out]
  n3619 = flat-sequence {
    tunnel: w307 -> [w5557]
    tunnel: w309 -> [w5558]
    tunnel: [w5556] -> w289
    tunnel: [w5555] -> w288
    tunnel: w272 -> [_]
    tunnel: w224 -> [_]
    tunnel: w140 -> [_]
    tunnel: w289 -> [w5559]
    tunnel: w288 -> [w5560]
    frame #0 {
      w5554 = FALSE ("AI to FIFO")
      n3620 = xnode "Read/Write Control"("FPGA VI Reference In"=w5558, "error in"=w5557, "AI to FIFO"=w5554, "APD to FIFO"=w5554) -> ("FPGA VI Reference Out"=w5556:T22, "error out"=w5555:errorcluster)
    }
    frame #1 {
      n3621 = xnode "Close FPGA VI Reference"("FPGA VI Reference In"=w5559, "error in"=w5560) -> ("error out"=→"error out":errorcluster)
    }
  }
